vi "UHR-Fleezers Control (host) - 12.7d.vi"() -> ()   [LabVIEW 2012] (continued)
            n859 = Multiply(x="Volume (uL) P3", y=w1280) -> (x*y=w1279:dbl)
            n860 = Concatenate Strings("tvolume  " ("string"), w1287, " u" ("string"), "\r") -> (w1285:string)
            n861 = Multiply(x=w1279, y=60.0) -> (x*y=→"HP3 Flush Time (s)":dbl)
            n862 = VISA Write(VISA resource name=w1296, write buffer=w1285) -> (VISA resource name out=w1284:refnum<visa-resource-name>)  [unwired: 1 in, 2 out]
            n863 = Concatenate Strings("cvolume" ("string"), "\r") -> (w1283:string)
            n864 = VISA Write(VISA resource name=w1284, write buffer=w1283) -> (VISA resource name out=w1294:refnum<visa-resource-name>)  [unwired: 1 in, 2 out]
            n865 = Concatenate Strings("irun" ("string"), "\r") -> (w1292:string)
            n866 = VISA Write(VISA resource name=w1294, write buffer=w1292) -> ()  [unwired: 1 in, 3 out]
          }
          frame #1 {
            "Flushing P3" <- TRUE ("Flushing P3")
          }
        }
      }
      event "Flush Pump 1": Value Change {
        n867 = event-data() -> ()  [unwired: 7 out]
        n868 = flat-sequence {
          tunnel: [w1314] -> w1304
          tunnel: w1303 -> [w1307]
          tunnel: w1304 -> [_]
          frame #0 {
            # "set paramaters (rate, volume) for flush, clear volume"
            n869 = local write "Inject Pump 1"(TRUE ("Inject Pump 1")) -> ()
            n870 = Number To Decimal String(number="Flush rate (uL/m) P1") -> (decimal integer string=w1330:string)  [unwired: 1 in]
            n871 = Concatenate Strings("irate  " ("string"), w1330, " u/m" ("string"), "\r") -> (w1332:string)
            n872 = VISA Write(VISA resource name=w1307, write buffer=w1332) -> (VISA resource name out=w1328:refnum<visa-resource-name>)  [unwired: 1 in, 2 out]
            n873 = Reciprocal(x="Flush rate (uL/m) P1") -> (1/x=w1311:dbl)
            n874 = Number To Decimal String(number="Volume (uL) P1") -> (decimal integer string=w1319:string)  [unwired: 1 in]
            n875 = Multiply(x="Volume (uL) P1", y=w1311) -> (x*y=w1310:dbl)
            n876 = Concatenate Strings("tvolume  " ("string"), w1319, " u" ("string"), "\r") -> (w1317:string)
            n877 = Multiply(x=w1310, y=60.0) -> (x*y=→"HP1 Flush Time (s)":dbl)
            n878 = VISA Write(VISA resource name=w1328, write buffer=w1317) -> (VISA resource name out=w1316:refnum<visa-resource-name>)  [unwired: 1 in, 2 out]
            n879 = Concatenate Strings("cvolume" ("string"), "\r") -> (w1315:string)
            n880 = VISA Write(VISA resource name=w1316, write buffer=w1315) -> (VISA resource name out=w1326:refnum<visa-resource-name>)  [unwired: 1 in, 2 out]
            n881 = Concatenate Strings("irun" ("string"), "\r") -> (w1324:string)
            n882 = VISA Write(VISA resource name=w1326, write buffer=w1324) -> (VISA resource name out=w1314:refnum<visa-resource-name>)  [unwired: 1 in, 2 out]
          }
          frame #1 {
            "Flushing P1" <- TRUE ("Flushing P3")
          }
        }
      }
      event "Clear Volume": Value Change {
        n883 = event-data() -> ()  [unwired: 7 out]
        n884 = Concatenate Strings("cvolume" ("string"), "\r") -> (w1336:string)
        n885 = VISA Write(VISA resource name=w1335, write buffer=w1336) -> ()  [unwired: 1 in, 3 out]
      }
      event "Clear Volume P3": Value Change {
        n886 = event-data() -> ()  [unwired: 7 out]
        n887 = Concatenate Strings("cvolume" ("string"), "\r") -> (w1342:string)
        n888 = VISA Write(VISA resource name=w1341, write buffer=w1342) -> ()  [unwired: 1 in, 3 out]
        n889 = local write "Clear Volume P3"(FALSE ("Clear Volume P3")) -> ()
      }
      event "Clear Volume P1": Value Change {
        n890 = event-data() -> ()  [unwired: 7 out]
        n891 = Concatenate Strings("cvolume" ("string"), "\r") -> (w1347:string)
        n892 = local write "Clear Volume P1"(FALSE ("Clear Volume P1")) -> ()
        n893 = VISA Write(VISA resource name=w1346, write buffer=w1347) -> ()  [unwired: 1 in, 3 out]
      }
      event "Display On P3": Value Change {
        n894 = event-data() -> ()  [unwired: 7 out]
        n895 = Select(t="dim 100", s="Display On P3", f="dim 0") -> (s? t:f=w1353:string)
        n896 = Concatenate Strings(w1353, "\r") -> (w1355:string)
        n897 = VISA Write(VISA resource name=w1350, write buffer=w1355) -> ()  [unwired: 1 in, 3 out]
      }
      event "Display On P1": Value Change {
        n898 = event-data() -> ()  [unwired: 7 out]
        n899 = Select(t="dim 100", s="Display On P1", f="dim 0") -> (s? t:f=w1360:string)
        n900 = Concatenate Strings(w1360, "\r") -> (w1362:string)
        n901 = VISA Write(VISA resource name=w1357, write buffer=w1362) -> ()  [unwired: 1 in, 3 out]
      }
      event "Retract Pump 3": Value Change {
        n902 = event-data() -> ()  [unwired: 7 out]
        n903 = local write "Retract Pump 3"(FALSE ("Retract Pump 3")) -> ()
        n904 = case shown="True" "Retract Pump 3" {
          tunnel: w1364 -> [_ w1367]
          frame False {
          }
          frame True {
            n905 = Number To Decimal String(number="Retract Rate (uL/m)") -> (decimal integer string=w1385:string)  [unwired: 1 in]
            n906 = Concatenate Strings("wrate  " ("string"), w1385, " u/m" ("string"), "\r") -> (w1387:string)
            n907 = VISA Write(VISA resource name=w1367, write buffer=w1387) -> (VISA resource name out=w1378:refnum<visa-resource-name>)  [unwired: 1 in, 2 out]
            n908 = Number To Decimal String(number="Retract Vol 3 (uL)") -> (decimal integer string=w1380:string)  [unwired: 1 in]
            n909 = Concatenate Strings("tvolume  " ("string"), w1380, " u" ("string"), "\r") -> (w1377:string)
            n910 = VISA Write(VISA resource name=w1378, write buffer=w1377) -> (VISA resource name out=w1373:refnum<visa-resource-name>)  [unwired: 1 in, 2 out]
            n911 = Concatenate Strings("cvolume" ("string"), "\r") -> (w1374:string)
            n912 = VISA Write(VISA resource name=w1373, write buffer=w1374) -> (VISA resource name out=w1368:refnum<visa-resource-name>)  [unwired: 1 in, 2 out]
            n913 = Concatenate Strings("wrun" ("string"), "\r") -> (w1369:string)
            n914 = VISA Write(VISA resource name=w1368, write buffer=w1369) -> ()  [unwired: 1 in, 3 out]
          }
        }
      }
      event "Retract Pump 1": Value Change {
        n915 = event-data() -> ()  [unwired: 7 out]
        n916 = local write "Retract Pump 1"(FALSE ("Retract Pump 1")) -> ()
        n917 = case shown="True" "Retract Pump 1" {
          tunnel: w1389 -> [_ w1394]
          frame False {
          }
          frame True {
            n918 = local read "Retract Rate (uL/m)"() -> (w1392:dbl)
            n919 = Number To Decimal String(number=w1392) -> (decimal integer string=w1410:string)  [unwired: 1 in]
            n920 = Concatenate Strings("wrate  " ("string"), w1410, " u/m" ("string"), "\r") -> (w1412:string)
            n921 = VISA Write(VISA resource name=w1394, write buffer=w1412) -> (VISA resource name out=w1404:refnum<visa-resource-name>)  [unwired: 1 in, 2 out]
            n922 = Number To Decimal String(number="Retract Vol 1 (uL)") -> (decimal integer string=w1406:string)  [unwired: 1 in]
            n923 = Concatenate Strings("tvolume  " ("string"), w1406, " u" ("string"), "\r") -> (w1403:string)
            n924 = VISA Write(VISA resource name=w1404, write buffer=w1403) -> (VISA resource name out=w1400:refnum<visa-resource-name>)  [unwired: 1 in, 2 out]
            n925 = Concatenate Strings("cvolume" ("string"), "\r") -> (w1401:string)
            n926 = VISA Write(VISA resource name=w1400, write buffer=w1401) -> (VISA resource name out=w1395:refnum<visa-resource-name>)  [unwired: 1 in, 2 out]
            n927 = Concatenate Strings("wrun" ("string"), "\r") -> (w1396:string)
            n928 = VISA Write(VISA resource name=w1395, write buffer=w1396) -> ()  [unwired: 1 in, 3 out]
          }
        }
      }
      event "Flip Green Filter": Value Change {
        n929 = event-data() -> ()  [unwired: 7 out]
        n930 = Not(x="Flip Green Filter") -> (.not. x?=w1415:bool)
        n931 = local write "Flip Green Filter"(w1415) -> ()
        n932 = flat-sequence {
          tunnel: [w1424] -> w1420
          tunnel: [w1423] -> w1419
          tunnel: w1414 -> [w1422]
          tunnel: [w1427] -> w1418
          tunnel: w1420 -> [w1427]
          tunnel: [w1426] -> w1417
          tunnel: w1419 -> [w1426]
          tunnel: w1418 -> [w1431]
          tunnel: w1417 -> [w1430]
          tunnel: [w1429] -> w1421
          frame #0 {
            n933 = xnode "Read/Write Control"("FPGA VI Reference In"=w1422, "Green Filter Flipper"=TRUE) -> ("FPGA VI Reference Out"=w1424:T20, "error out"=w1423:errorcluster)  [unwired: 1 in]
          }
          frame #1 {
            n934 = Wait (ms)(milliseconds to wait=u32 100) -> ()  [unwired: 1 out]
          }
          frame #2 {
            n935 = xnode "Read/Write Control"("FPGA VI Reference In"=w1431, "error in"=w1430, "Green Filter Flipper"=FALSE) -> ("error out"=w1429:errorcluster)  [unwired: 1 out]
          }
        }
      }
      event "Pump 1 contents", "Pump 3 contents": Value Change {
        n936 = event-data() -> ()  [unwired: 7 out]
        n937 = local read "Pump 1 contents"() -> (→"Pump 1 cont disp":string)
        n938 = local read "Pump 3 contents"() -> (→"Pump 3 cont disp":string)
      }
      event "Reset Trap Pos. FB": Value Change {
        n939 = event-data() -> ()  [unwired: 7 out]
        n940 = xnode "Read/Write Control"("FPGA VI Reference In"=w1435, "Trap Pos. FB Reset"="Reset Trap Pos. FB") -> ()  [unwired: 1 in, 2 out]
      }
      event "Rem fb disp offset": Value Change {
        n941 = event-data() -> ()  [unwired: 7 out]
        n942 = local write "Rem fb disp offset"(FALSE ("Rem fb disp offset")) -> ()
        n943 = local read "Mean T1 Position (nm)"() -> (w1438:dbl)
        n944 = local read "FB Trap Pos Offset"() -> (w1439:dbl)
        n945 = Subtract(x=w1439, y=w1438) -> (x-y=w1437:dbl)
        n946 = local write "FB Trap Pos Offset"(w1437) -> ()
      }
      event "Threshold (nm)": Value Change {
        n947 = event-data() -> ()  [unwired: 7 out]
        n948 = flat-sequence {
          tunnel: [w1444] -> w1442
          tunnel: w1441 -> [w1443]
          tunnel: w1442 -> [w1455]
          frame #0 {
            n949 = xnode "Read/Write Control"("FPGA VI Reference In"=w1443) -> ("FPGA VI Reference Out"=w1447:T20, "error out"=w1446:errorcluster, "FPGA TTrig Thresh"=w1448:i64)  [unwired: 1 in]
            n950 = local read "Threshold stored (nm)"() -> (w1454:dbl)
            n951 = local read "Threshold (nm)"() -> (w1444:dbl)
            n952 = local read "AOM X Cal (nm/MHz)"() -> (w1452:dbl)
            n953 = Subtract(x=w1444, y=w1454) -> (x-y=w1453:dbl)
            n954 = Divide(x=w1453, y=w1452) -> (x/y=w1450:dbl)
            n955 = call "IR AOM freq to word.vi"("Frequency In (MHz)"=w1450) -> ("Frequency Word Out (double)"=w1451:dbl)
            n956 = To Quad Integer(1:w1451) -> (0:w1449:i64)
            n957 = Add(x=w1448, y=w1449) -> (x+y=w1445:i64)
            n958 = xnode "Read/Write Control"("FPGA VI Reference In"=w1447, "error in"=w1446, "FPGA TTrig Thresh"=w1445) -> ()  [unwired: 2 out]
          }
          frame #1 {
            "Threshold stored (nm)" <- w1455
          }
        }
      }
      event "FB Trig Integrate": Value Change {
        n959 = event-data() -> ()  [unwired: 7 out]
        n960 = local read "FB Trig Integrate"() -> (w1458:u32)
        n961 = xnode "Read/Write Control"("FPGA VI Reference In"=w1456, "FB Trig Integrate"=w1458) -> ("error out"=w1457:errorcluster)  [unwired: 1 in, 1 out]
      }
      event "11": Value Change {
        n962 = event-data() -> ()  [unwired: 7 out]
        n963 = local read "11"() -> (w1459:bool)
        n964 = case shown="True" w1459 {
          frame False {
          }
          frame True {
            n965 = local read "Messages"() -> (w1461:string)
            n966 = call "Update messages.vi"("Message to add"="You kicked it up to 11!", "Old message string"=w1461) -> ("New message string"=w1462:string)
            n967 = call <vilib>:"Beep.vi"() -> ()  [unwired: 12 in]
            n968 = local write "Messages"(w1462) -> ()
          }
        }
      }
      event "Trap Pos. FB ON": Value Change {
        n969 = event-data() -> ()  [unwired: 7 out]
        n970 = xnode "Read/Write Control"("FPGA VI Reference In"=w1463, "Force feedback"="Trap Pos. FB ON") -> ()  [unwired: 1 in, 2 out]
      }
      event "Remove Action Offset": Value Change {
        n971 = event-data() -> ()  [unwired: 7 out]
        n972 = local write "Remove Action Offset"(FALSE ("Remove Action Offset")) -> ()
        n973 = local read "Trap Pos. FB Mult Factor"() -> (w1470:i64)
        n974 = local read "Trap Pos FB Action"() -> (w1468:i64)
        n975 = local read "Trap Pos. FB Offset Factor"() -> (w1466:i64)
        n976 = Multiply(x=w1470, y=w1468) -> (x*y=w1469:i64)
        n977 = Add(x=w1469, y=w1466) -> (x+y=w1467:i64)
        n978 = local write "Trap Pos. FB Offset Factor"(w1467) -> ()
        n979 = xnode "Read/Write Control"("FPGA VI Reference In"=w1465, "Trap Pos. FB Offset Factor"=w1467) -> ()  [unwired: 1 in, 2 out]
      }
      event "Remove Unwinding Offset": Value Change {
        n980 = event-data() -> ()  [unwired: 7 out]
        n981 = local write "Remove Unwinding Offset"(FALSE ("Remove Action Offset")) -> ()
        n982 = local read "Trap Pos. FB Mult Factor"() -> (w1484:i64)
        n983 = local read "Trap Pos FB Action"() -> (w1482:i64)
        n984 = local read "Trap Pos. FB Offset Factor"() -> (w1481:i64)
        n985 = Multiply(x=w1484, y=w1482) -> (x*y=w1483:i64)
        n986 = local read "Trap Pos. FB Mult Factor"() -> (w1480:i64)
        n987 = Add(x=w1483, y=w1481) -> (x+y=w1474:i64)
        n988 = Multiply(x=32768, y="factor") -> (x*y=w1477:dbl)
        n989 = Multiply(x=w1477, y=w1480) -> (x*y=w1479:dbl)
        n990 = Subtract(x=w1474, y=w1479) -> (x-y=w1478:dbl)
        n991 = To Quad Integer(1:w1478) -> (0:w1473:i64)
        n992 = xnode "Read/Write Control"("FPGA VI Reference In"=w1472, "Trap Pos. FB Offset Factor"=w1473) -> ()  [unwired: 1 in, 2 out]
        n993 = local write "Trap Pos. FB Offset Factor"(w1473) -> ()
      }
      event "Trap Pos. FB Range", "Trap Pos. FB Gains", "Trap Pos. FB Mult Factor", "Trap Pos. FB Offset Factor", "Trap Pos FB Negate Action", "Trap Pos FB Monitor\nT1 or T2", "Differential FB?", "Negate Diff?": Value Change {
        n994 = event-data() -> ()  [unwired: 7 out]
        n995 = Unbundle By Name("Trap Pos. FB Gains") -> ("proportional gain (Kc)"=w1489:fxp<+/-,16,8>, "integral gain (Kc*Ts/Ti)"=w1488:fxp<+/-,16,8>, "derivative gain (Kc*Td/Ts)"=w1487:fxp<+/-,16,8>)
        n996 = local read "Negate Diff?"() -> (w1494:bool)
        n997 = Unbundle By Name("Trap Pos. FB Range") -> ("output high"=w1492:fxp<+/-,16,1>, "output low"=w1491:fxp<+/-,16,1>)
        n998 = xnode "Read/Write Control"("FPGA VI Reference In"=w1486, "FB2 output high"=w1492, "FB2 output low"=w1491, "P2"=w1489, "I2"=w1488, "D2"=w1487, "Trap Pos. FB Mult Factor"="Trap Pos. FB Mult Factor", "Trap Pos. FB Offset Factor"="Trap Pos. FB Offset Factor", "Trap Pos FB Negate Action"="Trap Pos FB Negate Action", "Trap Pos FB Monitor T1 or T2"="Trap Pos FB Monitor\nT1 or T2", "AI1 X Scale"="Trap Pos. AI1 X Pre-scale", "Negate Diff?"=w1494, "Diff FB Measurement?"="Differential FB?") -> ()  [unwired: 1 in, 2 out]
      }
      event "Trap Pos FB SP", "Trap Pos FB SP 2", "Use SP 2": Value Change {
        n999 = event-data() -> ()  [unwired: 7 out]
        n1000 = Select(t="Trap Pos FB SP 2", s="Use SP 2", f="Trap Pos FB SP") -> (s? t:f=w1502:fxp<+/-,16,1>)
        n1001 = xnode "Read/Write Control"("FPGA VI Reference In"=w1501, "Trap Pos. FB SP"=w1502) -> ()  [unwired: 1 in, 2 out]
      }
      event "Offset SP2 from SP1": Value Change {
        n1002 = event-data() -> ()  [unwired: 7 out]
        n1003 = local read "Trap Pos FB SP"() -> (w1508:fxp<+/-,16,1>)
        n1004 = Add(x=w1508, y="SP2 Offset") -> (x+y=w1506:fxp<+/-,16,1>)
        n1005 = property on="Trap Pos FB SP 2" class="DigNum (strict)"("Val(Sgnl)"=w1506) -> ()  [unwired: 2 in, 2 out]
        n1006 = local write "Offset SP2 from SP1"(FALSE ("Offset SP2 from SP1")) -> ()
      }
      event "Set Reading to\nSetpoint": Value Change {
        # "This is the actual PID input signal"
        n1007 = event-data() -> ()  [unwired: 7 out]
        n1008 = local write "Set Reading to\nSetpoint"(FALSE ("Set SP to Reading")) -> ()
        n1009 = xnode "Read/Write Control"("FPGA VI Reference In"=w1510) -> ("FPGA VI Reference Out"=w1513:T20, "error out"=w1512:errorcluster, "Trap Pos FB Int-Norm Signal"=w1511:fxp<+/-,16,1>)  [unwired: 1 in]
        n1010 = local read "Differential FB?"() -> (w1514:bool)
        n1011 = case shown="False" w1514 {
          tunnel: [w1519 w1526] -> w1516
          tunnel: w1511 -> [w1517 w1526]
          frame False {
            n1012 = local read "Trap Pos FB Monitor\nT1 or T2"() -> (w1522:bool)
            n1013 = local read "Trap X AI1 (DMA)"() -> (w1525:T13)
            n1014 = Unbundle By Name(w1525) -> ("Set 1"=w1524:fxp<+/-,16,1>, "Set 2"=w1523:fxp<+/-,16,1>)
            n1015 = Select(t=w1524, s=w1522, f=w1523) -> (s? t:f=w1521:fxp<+/-,16,1>)
            n1016 = Not(x="Set SP Using...") -> (.not. x?=w1518:bool)
            n1017 = Select(t=w1517, s=w1518, f=w1521) -> (s? t:f=w1519:fxp<+/-,16,1>)
          }
          frame True {
          }
        }
        n1018 = xnode "Read/Write Control"("FPGA VI Reference In"=w1513, "error in"=w1512, "Trap Pos. FB SP"=w1516) -> ()  [unwired: 2 out]
        n1019 = local write "Trap Pos FB SP"(w1516) -> ()
      }
      event "Trap Pos. FB Out Scale 2^n": Value Change {
        n1020 = event-data() -> ()  [unwired: 7 out]
        n1021 = Scale By Power Of 2(n="Trap Pos. FB Out Scale 2^n", x=ext 1.0) -> (x*2^n=w1527:ext)
        n1022 = property on="Trap Pos. FB Mult Factor" class="DigNum (strict)"("Val(Sgnl)"=w1527) -> ()  [unwired: 2 in, 2 out]
      }
      event "Trap Pos FB Int Count": Value Change {
        n1023 = event-data() -> ()  [unwired: 7 out]
        n1024 = xnode "Read/Write Control"("FPGA VI Reference In"=w1530, "Trap Pos FB Int Count"="Trap Pos FB Int Count") -> ()  [unwired: 1 in, 2 out]
      }
      event "Trap pos": Value Change {
        n1025 = event-data() -> ()  [unwired: 7 out]
        n1026 = case shown="True" "Trap pos" {
          frame False {
            n1027 = property on="Trap Delta Graph" class="WFGraph (strict)"("Visible"=TRUE) -> ()  [unwired: 2 in, 2 out]
            n1028 = property on="Saved trap pos" class="WFGraph (strict)"("Visible"=FALSE) -> ()  [unwired: 2 in, 2 out]
          }
          frame True {
            n1029 = property on="Saved trap pos" class="WFGraph (strict)"("Visible"=TRUE) -> ()  [unwired: 2 in, 2 out]
            n1030 = property on="Trap Delta Graph" class="WFGraph (strict)"("Visible"=FALSE) -> ()  [unwired: 2 in, 2 out]
          }
        }
      }
    }
    "error out 2" <- w398
    n1031 = node-c288() -> ()  [unwired: 2 out]
  }
  n1032 = timed-loop "Rough control of MCL mirror stage (debugging)" {
    tunnel: [w1539] -> w76
    timing: w22 -> [_]
    timing-out: [_] -> w21
    tunnel: w5 -> [w1537]
    stop <- w1539 stop-if-true
    n1033 = node-c288() -> ()  [unwired: 2 out]
    n1034 = case shown="2" "MCL Mode" {
      tunnel: w1537 -> [_ w1542 w1589]
      frame 0, Default {
      }
      frame 1 {
        n1035 = node-c288() -> (w1544:T23)  [unwired: 4 out]
        n1036 = timed-loop "Oscillate MCL mirror" {
          timing: w1544 -> [_]
          timing-out: [_] -> w1543
          tunnel: w1542 -> [w1545]
          i -> [w1583]
          stop <- w1546 stop-if-true
          n1037 = node-c288() -> (w1582:i64)  [unwired: 1 out]
          n1038 = Multiply(x="AO1", y=32767.0) -> (x*y=w1578:dbl)
          n1039 = Multiply(x="AO2", y=32767.0) -> (x*y=w1573:dbl)
          n1040 = Divide(x=w1578, y=10.0) -> (x/y=w1579:dbl)
          n1041 = Divide(x=w1573, y=10.0) -> (x/y=w1574:dbl)
          n1042 = To Word Integer(number=w1579) -> (16bit integer=w1571:i16)
          n1043 = To Word Integer(number=w1574) -> (16bit integer=w1570:i16)
          n1044 = Divide(x=w1582, y=i64 1000) -> (x/y=w1553:dbl)
          n1045 = Multiply(x=w1553, y=w1583) -> (x*y=w1564:dbl)
          n1046 = Multiply(x="Osc. freq. (Hz) 2", y=6.283185307179586) -> (x*y=w1565:dbl)
          n1047 = Multiply(x=w1565, y=w1564) -> (x*y=w1563:dbl)
          n1048 = Sine(x=w1563) -> (sin(x)=w1562:dbl)
          n1049 = Multiply(x=w1562, y="Osc. amp. (V)") -> (x*y=w1560:dbl)
          n1050 = Add(x=w1560, y="Osc. center (V)") -> (x+y=w1558:dbl)
          n1051 = Divide(x=w1558, y=10.0) -> (x/y=w1556:dbl)
          n1052 = Multiply(x=w1556, y=32767.0) -> (x*y=w1551:dbl)
          n1053 = Select(t=w1551, s="Scan axis", f=w1571) -> (s? t:f=w1569:dbl)
          n1054 = Select(t=w1570, s="Scan axis", f=w1551) -> (s? t:f=w1568:dbl)
          n1055 = local read "MCL Mode"() -> (w1550:u16)
          n1056 = Not Equal?(x=w1550, y=u16 1) -> (x != y?=w1547:bool)
          n1057 = local read "Stop All"() -> (w1548:bool)
          n1058 = xnode "Read/Write Control"("FPGA VI Reference In"=w1545, "AO1"=w1569, "AO2"=w1568) -> ()  [unwired: 1 in, 2 out]
          n1059 = Compound Arithmetic op=OR(w1548, w1547) -> (w1546:bool)
          n1060 = node-c288() -> ()  [unwired: 2 out]
        }
        n1061 = node-c288(w1543) -> ()  [unwired: 1 out]
      }
      frame 2 {
        n1062 = case shown="True" "Start Scan" {
          tunnel: w1589 -> [_ w1591]
          frame False {
          }
          frame True {
            n1063 = Subtract(x="End (V)", y="Begin (V)") -> (x-y=w1598:dbl)
            n1064 = Decrement(x="N Points") -> (x-1=w1597:dbl)
            n1065 = Divide(x=w1598, y=w1597) -> (x/y=w1595:dbl)
            n1066 = for {
              N: "N Points" -> [_]
              tunnel: "Begin (V)" -> [w1614]
              tunnel: [w1606] -> w1601 mode=indexing
              tunnel: w1595 -> [w1605]
              tunnel: [w1603] -> w1594 mode=indexing
              tunnel: w1591 -> [w1602]
              i -> [w1613]
              n1067 = Multiply(x=w1605, y=w1613) -> (x*y=w1612:dbl)
              n1068 = Add(x=w1614, y=w1612) -> (x+y=w1609:dbl)
              n1069 = local read "Scan axis"() -> (w1604:bool)
              n1070 = local read "AO1"() -> (w1611:dbl)
              n1071 = local read "AO2"() -> (w1610:dbl)
              n1072 = Select(t=w1609, s=w1604, f=w1611) -> (s? t:f=w1608:dbl)
              n1073 = Select(t=w1610, s=w1604, f=w1609) -> (s? t:f=w1607:dbl)
              n1074 = flat-sequence {
                tunnel: w1608 -> [w1618]
                tunnel: w1607 -> [w1617]
                tunnel: w1602 -> [w1615]
                tunnel: [w1628] -> w1606
                tunnel: [w1627] -> w1603
                frame #0 {
                  w1621 = 10.0 ("y")
                  w1616 = 32767.0 ("y")
                  n1075 = Multiply(x=w1618, y=w1616) -> (x*y=w1624:dbl)
                  n1076 = Multiply(x=w1617, y=w1616) -> (x*y=w1622:dbl)
                  n1077 = Divide(x=w1624, y=w1621) -> (x/y=w1625:dbl)
                  n1078 = Divide(x=w1622, y=w1621) -> (x/y=w1623:dbl)
                  n1079 = To Word Integer(number=w1625) -> (16bit integer=w1619:i16)
                  n1080 = To Word Integer(number=w1623) -> (16bit integer=w1620:i16)
                  n1081 = xnode "Read/Write Control"("FPGA VI Reference In"=w1615, "AO1"=w1619, "AO2"=w1620) -> ()  [unwired: 1 in, 2 out]
                }
                frame #1 {
                  n1082 = Wait (ms)(milliseconds to wait="DAQ Delay (ms)") -> ()  [unwired: 1 out]
                }
                frame #2 {
                  n1083 = local read "Slow mean"() -> (w1628:dbl)
                  n1084 = local read "Sigma"() -> (w1627:dbl)
                }
              }
            }
            n1085 = Bundle("Begin (V)"="Begin (V)", w1595, w1601) -> (→"MCL Scan":cluster{"Begin (V)":dbl, dbl, dbl[]})  [unwired: 1 out]
            n1086 = Bundle("Begin (V)"="Begin (V)", w1595, w1594) -> (→"MCL Scan 2":cluster{"Begin (V)":dbl, dbl, dbl[]})  [unwired: 1 out]
          }
        }
      }
    }
    n1087 = local read "Stop All"() -> (w1539:bool)
    n1088 = node-c288() -> ()  [unwired: 2 out]
  }
  n1089 = timed-loop "Run Scripts, including: stage motion" {
    tunnel: w59 -> [w1637]
    tunnel: w58 -> [w1638]
    tunnel: [w1638] -> w57
    tunnel: [w1637] -> w56
    timing: w54 -> [_]
    timing-out: [_] -> w53
    tunnel: w42 -> [w1636]
    tunnel: w43 -> [w1635]
    tunnel: w32 -> [w1632]
    tunnel: w31 -> [w1631]
    tunnel: w30 -> [w1633]
    tunnel: w29 -> [w1634]
    tunnel: w17 -> [w1630]
    tunnel: w5 -> [w1629]
    stop <- w1639 stop-if-true
    n1090 = node-c288() -> ()  [unwired: 1 in, 1 out]
    n1091 = event shown="[22] \"Move in a Circle\": Value Change" {
      selector: _ -> [_ _ _ _ _ _ _ _ _ _ _ _ _ _ _ _ _ _ _ _ _ _ _ _]
      dyn-events: _ -> [_ _ _ _ _ _ _ _ _ _ _ _ _ _ _ _ _ _ _ _ _ _ _ _]
      timeout: _ -> [_ _ _ _ _ _ _ _ _ _ _ _ _ _ _ _ _ _ _ _ _ _ _ _]
      tunnel: ["Set Position" "Move to Position" _ _ _ _ _ _ "Read Harvard" _ _ _ _ _ _ "Got ADig bead" "Force FB Data\nScript" _ "Got DNA bead" "Take Stepping Data" _ "Take Detection Laser\nImage" _ _] -> _
      tunnel: [_ _ _ _ _ _ _ _ _ _ _ _ _ _ _ _ _ _ _ _ _ _ _ w2453] -> w1639
      tunnel: w1637 -> [w1657 w1665 w1678 w1708 _ _ _ _ _ w1824 w1864 w1945 w1974 w2106 w2132 _ w2168 _ _ _ _ _ _ _]
      tunnel: w1638 -> [w1658 w1666 w1679 w1709 _ _ _ _ _ w1825 w1865 w1946 w1975 w2107 w2133 _ w2169 _ _ _ _ _ _ _]
      tunnel: w1636 -> [_ _ _ _ _ _ _ _ w1809 _ _ _ _ _ _ _ _ _ _ _ _ _ _ _]
      tunnel: w1635 -> [_ _ _ _ _ _ _ _ w1808 _ _ _ _ _ _ _ _ _ _ _ _ _ _ _]
      tunnel: w1634 -> [_ _ _ _ _ _ _ _ _ _ _ _ _ _ _ _ _ _ _ _ _ _ _ _]
      tunnel: w1633 -> [_ _ _ _ _ _ _ _ _ _ _ _ _ _ _ _ _ _ _ _ _ _ _ _]
      tunnel: w1632 -> [_ _ _ _ _ _ _ _ _ _ _ _ _ _ _ _ _ _ _ _ _ _ _ _]
      tunnel: w1631 -> [_ _ _ _ _ _ _ _ _ _ _ _ _ _ _ _ _ _ _ _ _ _ _ _]
      tunnel: w1630 -> [_ _ _ _ w1736 w1764 w1788 w1799 _ _ _ _ _ _ _ _ _ _ _ _ _ _ _ w2452]
      tunnel: w1629 -> [_ _ _ _ _ _ _ _ _ _ _ _ _ _ _ _ _ _ _ _ _ _ w2328 _]
      event "Set Position", "Set Position 2", "Set Position 3", "Set Position 4", "Set Position 5", "Set Position 1": Value Change {
        n1092 = event-data() -> ()  [unwired: 1 in, 5 out]
        n1093 = Build Array("Set Position 1", "Set Position 2", "Set Position 3", "Set Position 4", "Set Position 5") -> (w1656:bool[])
        n1094 = Boolean Array To Number(Boolean array=w1656) -> (number=w1655:u32)
        n1095 = Logarithm Base 2(1:w1655) -> (0:w1647:dbl)
        n1096 = call "Read Stage Position.vi"("error in"=w1657, "VISA resource name in"=w1658) -> ("Current Position"=w1662:cluster{dbl, dbl, dbl}, "error out"=w1661:errorcluster)  [unwired: 2 out]
        n1097 = Decrement(x="Position") -> (x-1=w1645:dbl)
        n1098 = Greater Or Equal?(x=w1647, y=0.0) -> (x >= y?=w1648:bool)
        n1099 = Cluster To Array(cluster=w1662) -> (array=w1659:dbl[])
        n1100 = local write "Stage Control Serial Error"(w1661) -> ()
        n1101 = Select(t=w1647, s=w1648, f=w1645) -> (s? t:f=w1644:dbl)
        n1102 = Increment(x=w1644) -> (x+1=w1643:dbl)
        n1103 = Build Array (concatenate)(w1643, w1659) -> (w1642:dbl[])
        n1104 = Replace Array Subset(array="Saved Stage Positions", new element=w1642, index (row)=w1644) -> (w1660:dbl[][])  [unwired: 1 in]
        n1105 = local write "Saved Stage Positions"(w1660) -> ()
      }
      event "Move to Position": Value Change {
        n1106 = event-data() -> ()  [unwired: 1 in, 5 out]
        n1107 = flat-sequence {
          tunnel: w1666 -> [w1670]
          tunnel: w1665 -> [w1669]
          frame #0 {
            n1108 = local read "Saved Stage Positions"() -> (w1672:dbl[][])
            n1109 = local read "Position"() -> (w1671:dbl)
            n1110 = local write "Stage Moving"(TRUE ("Stage Moving")) -> ()
            n1111 = call "move to saved stage position.vi"("error in"=w1669, "Stage VISA resource name in"=w1670, "Position"=w1671, "Saved Stage Positions"=w1672) -> ("error out"=w1668:errorcluster)  [unwired: 1 out]
            n1112 = local write "Stage Control Serial Error"(w1668) -> ()
          }
          frame #1 {
            n1113 = call <vilib>:"Beep.vi"() -> ()  [unwired: 3 in, 9 out]
            n1114 = local write "Stage Moving"(FALSE ("Stage Moving")) -> ()
          }
        }
      }
      event "Move Cap. 1 (DNA Bottom)": Value Change {
        n1115 = event-data() -> ()  [unwired: 1 in, 5 out]
        n1116 = local write "Move Cap. 1 (DNA Bottom)"(FALSE ("Move Cap. 1 (DNA Right)")) -> ()
        n1117 = flat-sequence {
          tunnel: w1678 -> [w1681]
          tunnel: w1679 -> [w1682]
          tunnel: [w1682] -> w1676
          tunnel: [w1681] -> w1675
          tunnel: w1676 -> [w1684]
          tunnel: w1675 -> [w1683]
          frame #0 {
            n1118 = property on="Sample Channel\nFlow" class="Bool (strict)"("Val(Sgnl)"="Cap 1 Samp Flow ON") -> ()  [unwired: 2 in, 2 out]
          }
          frame #1 {
            n1119 = local read "Saved Stage Positions"() -> (w1694:dbl[][])
            n1120 = local write "Stage Moving"(TRUE ("Stage Moving")) -> ()
            n1121 = Array Subset(array=w1694, index (row)=0 ("index"), length (row)=1 ("length"), index (col)=1 ("index"), length (col)=3 ("length")) -> (w1691:dbl[][])
            n1122 = Reshape Array(w1691, 3 ("dimension size")) -> (w1689:dbl[])
            n1123 = Array To Cluster(array=w1689) -> (cluster=w1688:cluster{"[0]":dbl, "[1]":dbl, "[2]":dbl})
            n1124 = call "Set Stage Position.vi"("Position"=w1688, "error in"=w1683, "VISA resource name in"=w1684) -> ("error out"=w1687:errorcluster)  [unwired: 2 out]
            n1125 = local write "Stage Control Serial Error"(w1687) -> ()
          }
          frame #2 {
            n1126 = local write "Stage Moving"(FALSE ("Stage Moving")) -> ()
            n1127 = case shown="True" "Cap 1 Flow ON" {
              frame False {
              }
              frame True {
                n1128 = property on="Inject Pump 1" class="Bool (strict)"("Val(Sgnl)"=TRUE ("Value (Signaling)")) -> ()  [unwired: 2 in, 2 out]
              }
            }
            n1129 = call <vilib>:"Beep.vi"() -> ()  [unwired: 3 in, 9 out]
          }
          frame #3 {
            n1130 = property on="Sample Channel\nFlow" class="Bool (strict)"("Val(Sgnl)"=FALSE ("Value (Signaling)")) -> ()  [unwired: 2 in, 2 out]
            n1131 = local read "Cap. 2 BD T1?\n(ADig T1, DNA T2)"() -> (w1701:bool)
            n1132 = case shown="True" w1701 {
              tunnel: "Cap 1 T ON" -> [w1703 w1704]
              frame False {
                n1133 = property on="Trap 1 (ON/OFF)" class="Bool (strict)"("Val(Sgnl)"=w1703) -> ()  [unwired: 2 in, 2 out]
              }
              frame True {
                n1134 = property on="Trap 2 (ON/OFF)" class="Bool (strict)"("Val(Sgnl)"=w1704) -> ()  [unwired: 2 in, 2 out]
              }
            }
            n1135 = property on="Got DNA bead" class="Bool"("Key Focus"=TRUE) -> ()  [unwired: 2 in, 2 out]
          }
        }
      }
      event "Move Cap. 2 (ADig Top)": Value Change {
        n1136 = event-data() -> ()  [unwired: 1 in, 5 out]
        n1137 = local write "Move Cap. 2 (ADig Top)"(FALSE ("Move Cap. 2 (ADig Left)")) -> ()
        n1138 = flat-sequence {
          tunnel: w1708 -> [w1711]
          tunnel: w1709 -> [w1712]
          tunnel: [w1712] -> w1706
          tunnel: [w1711] -> w1705
          tunnel: w1706 -> [w1715]
          tunnel: w1705 -> [w1714]
          frame #0 {
            n1139 = property on="Sample Channel\nFlow" class="Bool (strict)"("Val(Sgnl)"="Cap 2 Samp Flow ON") -> ()  [unwired: 2 in, 2 out]
          }
          frame #1 {
            w1713 = FALSE ("Value (Signaling)")
            n1140 = local read "Saved Stage Positions"() -> (w1725:dbl[][])
            n1141 = local write "Stage Moving"(TRUE ("Stage Moving")) -> ()
            n1142 = Array Subset(array=w1725, index (row)=1 ("index"), length (row)=1 ("length"), index (col)=1 ("index"), length (col)=3 ("length")) -> (w1722:dbl[][])
            n1143 = Reshape Array(w1722, 3 ("dimension size")) -> (w1720:dbl[])
            n1144 = property on="Trap 1 (ON/OFF)" class="Bool (strict)"("Val(Sgnl)"=w1713) -> ()  [unwired: 2 in, 2 out]
            n1145 = property on="Trap 1 (ON/OFF)" class="Bool (strict)"("Val(Sgnl)"=w1713) -> ()  [unwired: 2 in, 2 out]
            n1146 = Array To Cluster(array=w1720) -> (cluster=w1719:cluster{"[0]":dbl, "[1]":dbl, "[2]":dbl})
            n1147 = call "Set Stage Position.vi"("Position"=w1719, "error in"=w1714, "VISA resource name in"=w1715) -> ("error out"=w1718:errorcluster)  [unwired: 2 out]
            n1148 = local write "Stage Control Serial Error"(w1718) -> ()
          }
          frame #2 {
            n1149 = local write "Stage Moving"(FALSE ("Stage Moving")) -> ()
            n1150 = call <vilib>:"Beep.vi"() -> ()  [unwired: 3 in, 9 out]
            n1151 = case shown="True" "Cap 2 Flow ON" {
              frame False {
              }
              frame True {
                n1152 = property on="Inject Pump 3" class="Bool (strict)"("Val(Sgnl)"=TRUE ("Value (Signaling)")) -> ()  [unwired: 2 in, 2 out]
              }
            }
          }
          frame #3 {
            n1153 = property on="Sample Channel\nFlow" class="Bool (strict)"("Val(Sgnl)"=FALSE ("Value (Signaling)")) -> ()  [unwired: 2 in, 2 out]
            n1154 = case shown="False" "Cap. 2 BD T1?\n(ADig T1, DNA T2)" {
              tunnel: "Cap 2 T ON" -> [w1734 w1735]
              frame False {
                n1155 = property on="Trap 2 (ON/OFF)" class="Bool (strict)"("Val(Sgnl)"=w1734) -> ()  [unwired: 2 in, 2 out]
              }
              frame True {
                n1156 = property on="Trap 1 (ON/OFF)" class="Bool (strict)"("Val(Sgnl)"=w1735) -> ()  [unwired: 2 in, 2 out]
              }
            }
            n1157 = property on="Got ADig bead" class="Bool"("Key Focus"=TRUE) -> ()  [unwired: 2 in, 2 out]
          }
        }
      }
      event "Initialize Blue Laser": Value Change {
        n1158 = event-data() -> ()  [unwired: 1 in, 5 out]
        n1159 = flat-sequence {
          tunnel: w1736 -> [w1755]
          frame #0 {
            n1160 = Concatenate Strings("slmp ", "Blue Laser\nModulation\nPower (mW)") -> (w1754:string)
            n1161 = call "serial write macro.vi"("String"=w1754, "Delay (ms)"="Delay (ms)", "VISA resource name"=w1755) -> ("read buffer"=w1743:string, "error out"=w1744:errorcluster, "VISA resource name out"=w1751:refnum<visa-resource-name>)
            n1162 = local write "read blue buffer"(w1743) -> ()
            n1163 = local write "Blue Error Out"(w1744) -> ()
            n1164 = call "serial write macro.vi"("String"="sdmes 1", "Delay (ms)"="Delay (ms)", "VISA resource name"=w1751) -> ("read buffer"=w1741:string, "error out"=w1742:errorcluster, "VISA resource name out"=w1749:refnum<visa-resource-name>)
            n1165 = local write "Blue Error Out"(w1742) -> ()
            n1166 = local write "read blue buffer"(w1741) -> ()
            n1167 = call "serial write macro.vi"("String"="sames 1", "Delay (ms)"="Delay (ms)", "VISA resource name"=w1749) -> ("read buffer"=w1738:string, "error out"=w1740:errorcluster, "VISA resource name out"=w1746:refnum<visa-resource-name>)
            n1168 = local write "read blue buffer"(w1738) -> ()
            n1169 = local write "Blue Error Out"(w1740) -> ()
            n1170 = call "serial write macro.vi"("String"="l1", "Delay (ms)"="Delay (ms)", "VISA resource name"=w1746) -> ("read buffer"=w1737:string, "error out"=w1739:errorcluster)  [unwired: 1 out]
            n1171 = local write "read blue buffer"(w1737) -> ()
            n1172 = local write "Blue Error Out"(w1739) -> ()
          }
          frame #1 {
            n1173 = local write "Initialize Blue Laser"(FALSE ("Initialize")) -> ()
          }
        }
      }
      event "Blue Laser Modluation Mode": Value Change {
        # "Changes the type of modulation for the blue laser"
        n1174 = event-data() -> ()  [unwired: 1 in, 5 out]
        n1175 = case shown="\"Constant Power\"" "Blue Laser Modluation Mode" {
          tunnel: ["sdmes 1" w1773 "sdmes 1" "sdmes 0"] -> w1758
          tunnel: ["sames 1" "cp" "sames 0" "sames 1"] -> w1757
          frame "Digital + Analog", Default {
          }
          frame "Constant Power" {
            n1176 = local read "Blue Laser\nModulation\nPower (mW)"() -> (w1776:string)
            n1177 = Decimal String To Number(string=w1776) -> (number=w1772:i32)  [unwired: 2 in, 1 out]
            n1178 = Divide(x=w1772, y=1000) -> (x/y=w1770:dbl)
            n1179 = Number To Fractional String(number=w1770) -> (F-format string=w1771:string)  [unwired: 3 in]
            n1180 = Concatenate Strings("p ", w1771) -> (w1773:string)
          }
          frame "Digital Only" {
          }
          frame "Analog Only" {
          }
        }
        n1181 = local read "Delay (ms)"() -> (w1767:i32)
        n1182 = call "serial write macro.vi"("String"=w1758, "Delay (ms)"=w1767, "VISA resource name"=w1764) -> ("read buffer"=w1765:string, "error out"=w1766:errorcluster, "VISA resource name out"=w1759:refnum<visa-resource-name>)
        n1183 = local write "read blue buffer"(w1765) -> ()
        n1184 = local write "Blue Error Out"(w1766) -> ()
        n1185 = local read "Delay (ms)"() -> (w1762:i32)
        n1186 = call "serial write macro.vi"("String"=w1757, "Delay (ms)"=w1762, "VISA resource name"=w1759) -> ("read buffer"=w1760:string, "error out"=w1761:errorcluster)  [unwired: 1 out]
        n1187 = local write "Blue Error Out"(w1761) -> ()
        n1188 = local write "read blue buffer"(w1760) -> ()
      }
      event "Blue Laser\nModulation\nPower (mW)": Value Change {
        n1189 = event-data() -> ()  [unwired: 1 in, 5 out]
        n1190 = local read "Blue Laser\nModulation\nPower (mW)"() -> (w1783:string)
        n1191 = local read "Blue Laser Modluation Mode"() -> (w1784:string)
        n1192 = case shown="\"Constant Power\"" w1784 {
          tunnel: w1783 -> [w1790 w1797]
          tunnel: [w1789 w1796] -> w1782
          frame "Constant Power" {
            # "Different command to change constant power instead of modulation power"
            n1193 = Decimal String To Number(string=w1790) -> (offset past number=w1795:i32)  [unwired: 2 in, 1 out]
            n1194 = Divide(x=w1795, y=1000) -> (x/y=w1793:dbl)
            n1195 = Number To Fractional String(number=w1793) -> (F-format string=w1791:string)  [unwired: 3 in]
            n1196 = Concatenate Strings("p ", w1791) -> (w1789:string)
          }
          frame Default {
            n1197 = Concatenate Strings("slmp ", w1797) -> (w1796:string)
          }
        }
        n1198 = local read "Delay (ms)"() -> (w1787:i32)
        n1199 = call "serial write macro.vi"("String"=w1782, "Delay (ms)"=w1787, "VISA resource name"=w1788) -> ("read buffer"=w1786:string, "error out"=w1785:errorcluster)  [unwired: 1 out]
        n1200 = local write "Blue Error Out"(w1785) -> ()
        n1201 = local write "read blue buffer"(w1786) -> ()
      }
      event "Send string\nto Blue Laser": Value Change {
        n1202 = event-data() -> ()  [unwired: 1 in, 5 out]
        n1203 = flat-sequence {
          tunnel: w1799 -> [w1804]
          frame #0 {
            n1204 = local read "Delay (ms)"() -> (w1801:i32)
            n1205 = call "serial write macro.vi"("String"="command string", "Delay (ms)"=w1801, "VISA resource name"=w1804) -> ("read buffer"=w1802:string, "error out"=→"Blue Error Out":errorcluster)  [unwired: 1 out]
            "read blue buffer" <- w1802
            n1206 = String Length(string=w1802) -> (length=→"length":i32)
            "command string sent" <- "command string"
          }
          frame #1 {
            n1207 = local write "Send string\nto Blue Laser"(FALSE ("Send string")) -> ()
          }
        }
      }
      event "Read Harvard": Value Change {
        n1208 = event-data() -> ()  [unwired: 1 in, 5 out]
        n1209 = Concatenate Strings("write buffer", "\r") -> (w1811:string)
        n1210 = VISA Write(VISA resource name=w1809, write buffer=w1811, error in (no error)=w1808) -> (VISA resource name out=w1820:refnum<visa-resource-name>, error out=w1819:errorcluster)  [unwired: 1 out]
        n1211 = stacked-sequence {
          tunnel: [w1823] -> w1818
          tunnel: w1820 -> [w1823]
          tunnel: w1819 -> [w1822]
          tunnel: [w1822] -> w1813
          frame #0 {
            n1212 = Wait (ms)(milliseconds to wait=50) -> ()  [unwired: 1 out]
          }
        }
        n1213 = property class="Instr"(reference=w1818, error in=w1813) -> (reference out=w1817:refnum<visa-resource-name>, error out=w1815:errorcluster, "Serial Settings:Number of Bytes at Serial Port"=w1816:u32)
        "Serial Settings:Number of Bytes at Serial Port" <- w1816
        n1214 = VISA Read(VISA resource name=w1817, byte count=w1816, error in (no error)=w1815) -> (read buffer=w1814:string)  [unwired: 3 out]
        "read buffer" <- w1814
        n1215 = Fract/Exp String To Number(string=w1814) -> ()  [unwired: 5 out]
      }
      event "+z", "-z": Value Change {
        n1216 = event-data() -> ()  [unwired: 1 in, 5 out]
        n1217 = flat-sequence {
          tunnel: w1824 -> [w1846]
          tunnel: w1825 -> [w1826]
          frame #0 {
            n1218 = call "Read Stage Position.vi"("error in"=w1846, "VISA resource name in"=w1826) -> ("Current Position"=w1831:cluster{dbl, dbl, dbl}, "error out"=w1844:errorcluster, "VISA resource name out"=w1845:refnum<visa-resource-name>)  [unwired: 1 out]
            n1219 = local read "Saved Stage Positions"() -> (w1855:dbl[][])
            n1220 = Divide(x="z nudge increment (um)", y=1000.0) -> (x/y=w1843:dbl)
            n1221 = Boolean To (0,1)(Boolean="+z") -> (0, 1=w1835:i16)
            n1222 = Boolean To (0,1)(Boolean="-z") -> (0, 1=w1836:i16)
            n1223 = Array Subset(array=w1855, index (row)=1 ("index"), length (row)=1 ("length"), index (col)=1 ("index"), length (col)=3 ("length")) -> (w1852:dbl[][])
            n1224 = Multiply(x=w1835, y=w1843) -> (x*y=w1839:dbl)
            n1225 = Multiply(x=w1836, y=w1843) -> (x*y=w1837:dbl)
            n1226 = Unbundle(w1831) -> (w1829:dbl, w1828:dbl, w1832:dbl)
            n1227 = Negate(x=w1837) -> (-x=w1838:dbl)
            n1228 = Reshape Array(w1852, 3 ("dimension size")) -> (w1850:dbl[])
            n1229 = Add(x=w1839, y=w1838) -> (x+y=w1840:dbl)
            n1230 = Array To Cluster(array=w1850) -> ()  [unwired: 1 out]
            n1231 = Add(x=w1840, y=w1832) -> (x+y=w1830:dbl)
            n1232 = Bundle(cluster=w1831, w1829, w1828, w1830) -> (w1827:cluster{dbl, dbl, dbl})
            n1233 = call "Set Stage Position.vi"("Position"=w1827, "error in"=w1844, "VISA resource name in"=w1845) -> ("error out"=w1849:errorcluster)  [unwired: 2 out]
            n1234 = local write "Stage Moving"(TRUE ("Stage Moving")) -> ()
            n1235 = local write "Stage Control Serial Error"(w1849) -> ()
          }
          frame #1 {
            n1236 = local write "Stage Moving"(FALSE ("Stage Moving")) -> ()
            n1237 = call <vilib>:"Beep.vi"() -> ()  [unwired: 3 in, 9 out]
          }
        }
      }
      event "Cal/Data Acq. Spot": Value Change {
        n1238 = event-data() -> ()  [unwired: 1 in, 5 out]
        n1239 = flat-sequence {
          tunnel: w1864 -> [w1868]
          tunnel: w1865 -> [w1869]
          tunnel: [w1869] -> w1861
          tunnel: [w1868] -> w1860
          tunnel: w1861 -> [w1874]
          tunnel: w1860 -> [w1873]
          tunnel: ["Cal @ (MHz)"] -> w1858
          tunnel: [w1878] -> w1862
          tunnel: w1858 -> [w1878]
          tunnel: w1862 -> [w1887]
          tunnel: ["W/ Offset 1"] -> w1859
          tunnel: w1862 -> [w1908]
          tunnel: w1859 -> [w1906]
          frame #0 {
            n1240 = property on="Sample Channel\nFlow" class="Bool (strict)"("Val(Sgnl)"="Daq spot flow on") -> ()  [unwired: 2 in, 2 out]
            n1241 = Wait (ms)(milliseconds to wait=u32 250) -> ()  [unwired: 1 out]
          }
          frame #1 {
            n1242 = local read "Saved Stage Positions"() -> (w1871:dbl[][])
            n1243 = property on="Trap Delta (MHz)" class="DigNum (strict)"("Val(Sgnl)"="Cal @ (MHz)") -> ()  [unwired: 2 in, 2 out]
            n1244 = local write "Stage Moving"(TRUE ("Stage Moving")) -> ()
            n1245 = call "move to saved stage position.vi"("error in"=w1873, "Stage VISA resource name in"=w1874, "Position"="Cal Stage Position", "Saved Stage Positions"=w1871) -> ("error out"=w1872:errorcluster)  [unwired: 1 out]
            n1246 = local write "Stage Control Serial Error"(w1872) -> ()
          }
          frame #2 {
            n1247 = local write "Stage Moving"(FALSE ("Stage Moving")) -> ()
            n1248 = property on="Sample Channel\nFlow" class="Bool (strict)"("Val(Sgnl)"="Flow ON during cal?") -> ()  [unwired: 2 in, 2 out]
            n1249 = call <vilib>:"Beep.vi"() -> ()  [unwired: 3 in, 9 out]
          }
          frame #3 {
            n1250 = Wait (ms)(milliseconds to wait=u32 1000) -> ()  [unwired: 1 out]
          }
          frame #4 {
            n1251 = property on="Save Calibration" class="Bool (strict)"("Val(Sgnl)"=TRUE ("Value (Signaling)")) -> ()  [unwired: 2 in, 2 out]
          }
          frame #5 {
            n1252 = Wait (ms)(milliseconds to wait=u32 2000) -> ()  [unwired: 1 out]
          }
          frame #6 {
            # "Check to see if \nsaving done"
            n1253 = while {
              stop <- w1883 stop-if-true
              n1254 = local read "Saving..."() -> (w1884:bool)
              n1255 = Wait (ms)(milliseconds to wait=u32 100) -> ()  [unwired: 1 out]
              n1256 = Not(x=w1884) -> (.not. x?=w1883:bool)
            }
          }
          frame #7 {
            n1257 = case shown="True" "W/ Offset 1" {
              tunnel: w1887 -> [_ w1888]
              frame False {
              }
              frame True {
                n1258 = stacked-sequence {
                  tunnel: w1888 -> [_ _ _ _ _ _ _ w1905]
                  frame #0 {
                    n1259 = property on="Trap Delta (MHz)" class="DigNum (strict)"("Val(Sgnl)"="Offset 1 Start (MHz)") -> ()  [unwired: 2 in, 2 out]
                    n1260 = Replace Array Subset(array=u32[] [0] ("Index Values"), new element="Offset 1 Set", index=0) -> (w1889:u32[])
                    n1261 = property on="Saved AOD Raster Scan Parameter Sets" class="Arr (strict)"("Index Values"=w1889) -> ()  [unwired: 2 in, 2 out]
                  }
                  frame #1 {
                    n1262 = Wait (ms)(milliseconds to wait=u32 200) -> ()  [unwired: 1 out]
                  }
                  frame #2 {
                    n1263 = property on="Load parameters" class="Bool (strict)"("Val(Sgnl)"=TRUE ("Value (Signaling)")) -> ()  [unwired: 2 in, 2 out]
                  }
                  frame #3 {
                    n1264 = Wait (ms)(milliseconds to wait=u32 200) -> ()  [unwired: 1 out]
                  }
                  frame #4 {
                    n1265 = property on="Trap Raster Scan" class="Bool (strict)"("Val(Sgnl)"=TRUE ("Value (Signaling)")) -> ()  [unwired: 2 in, 2 out]
                  }
                  frame #5 {
                    n1266 = Wait (ms)(milliseconds to wait=u32 2000) -> ()  [unwired: 1 out]
                  }
                  frame #6 {
                    n1267 = while {
                      stop <- w1902 stop-if-true
                      n1268 = local read "Raster Scanning..."() -> (w1904:bool)
                      n1269 = local read "Saving..."() -> (w1900:bool)
                      n1270 = Wait (ms)(milliseconds to wait=u32 100) -> ()  [unwired: 1 out]
                      n1271 = Not(x=w1900) -> (.not. x?=w1899:bool)
                      n1272 = Not(x=w1904) -> (.not. x?=w1901:bool)
                      n1273 = And(x=w1901, y=w1899) -> (x .and. y?=w1902:bool)
                    }
                  }
                  frame #7 {
                    n1274 = property on="Trap Delta (MHz)" class="DigNum (strict)"("Val(Sgnl)"=w1905) -> ()  [unwired: 2 in, 2 out]
                  }
                }
              }
            }
          }
          frame #8 {
            n1275 = local read "Save ave N"() -> (w1907:dbl)
            n1276 = case shown="False" "W/ Offset 2" {
              tunnel: w1908 -> [_ w1915]
              tunnel: w1907 -> [_ w1914]
              tunnel: w1906 -> [w1910 _]
              frame False {
                n1277 = case shown="False" w1910 {
                  frame False {
                    n1278 = Multiply(x="Cal read wait (s)", y=u32 1000 ("milliseconds to wait")) -> (x*y=w1912:u32)
                    n1279 = Wait (ms)(milliseconds to wait=w1912) -> ()  [unwired: 1 out]
                  }
                  frame True {
                  }
                }
              }
              frame True {
                n1280 = stacked-sequence {
                  tunnel: w1915 -> [_ _ _ _ _ _ _ _ _ w1936 _ _]
                  tunnel: w1914 -> [_ _ _ _ _ _ _ _ _ w1934 _ _]
                  frame #0 {
                    n1281 = property on="Save ave N" class="DigNum (strict)"("Val(Sgnl)"=1.0 ("Value (Signaling)")) -> ()  [unwired: 2 in, 2 out]
                  }
                  frame #1 {
                    n1282 = Wait (ms)(milliseconds to wait=u32 500) -> ()  [unwired: 1 out]
                  }
                  frame #2 {
                    n1283 = property on="Trap Delta (MHz)" class="DigNum (strict)"("Val(Sgnl)"="Offset 2 Start (MHz)") -> ()  [unwired: 2 in, 2 out]
                    n1284 = Replace Array Subset(array=u32[] [0] ("Index Values"), new element="Offset 2 Set", index=0) -> (w1920:u32[])
                    n1285 = property on="Saved AOD Raster Scan Parameter Sets" class="Arr (strict)"("Index Values"=w1920) -> ()  [unwired: 2 in, 2 out]
                  }
                  frame #3 {
                    n1286 = Wait (ms)(milliseconds to wait=u32 500) -> ()  [unwired: 1 out]
                  }
                  frame #4 {
                    n1287 = property on="Load parameters" class="Bool (strict)"("Val(Sgnl)"=TRUE ("Value (Signaling)")) -> ()  [unwired: 2 in, 2 out]
                  }
                  frame #5 {
                    n1288 = Wait (ms)(milliseconds to wait=u32 500) -> ()  [unwired: 1 out]
                  }
                  frame #6 {
                    n1289 = property on="Trap Raster Scan" class="Bool (strict)"("Val(Sgnl)"=TRUE ("Value (Signaling)")) -> ()  [unwired: 2 in, 2 out]
                  }
                  frame #7 {
                    n1290 = Wait (ms)(milliseconds to wait=u32 2000) -> ()  [unwired: 1 out]
                  }
                  frame #8 {
                    n1291 = while {
                      stop <- w1929 stop-if-true
                      n1292 = local read "Raster Scanning..."() -> (w1932:bool)
                      n1293 = local read "Saving..."() -> (w1930:bool)
                      n1294 = Wait (ms)(milliseconds to wait=u32 100) -> ()  [unwired: 1 out]
                      n1295 = Not(x=w1930) -> (.not. x?=w1928:bool)
                      n1296 = Not(x=w1932) -> (.not. x?=w1931:bool)
                      n1297 = And(x=w1931, y=w1928) -> (x .and. y?=w1929:bool)
                    }
                  }
                  frame #9 {
                    n1298 = property on="Trap Delta (MHz)" class="DigNum (strict)"("Val(Sgnl)"=w1936) -> ()  [unwired: 2 in, 2 out]
                    n1299 = property on="Saved AOD Raster Scan Parameter Sets" class="Arr (strict)"("Index Values"=u32[] [0]) -> ()  [unwired: 2 in, 2 out]
                    n1300 = property on="Save ave N" class="DigNum (strict)"("Val(Sgnl)"=w1934) -> ()  [unwired: 2 in, 2 out]
                  }
                  frame #10 {
                    n1301 = Wait (ms)(milliseconds to wait=u32 500) -> ()  [unwired: 1 out]
                  }
                  frame #11 {
                    n1302 = property on="Load parameters" class="Bool (strict)"("Val(Sgnl)"=TRUE ("Value (Signaling)")) -> ()  [unwired: 2 in, 2 out]
                  }
                }
              }
            }
          }
          frame #9 {
            n1303 = property on="Read Cal" class="Bool (strict)"("Val(Sgnl)"=TRUE ("Value (Signaling)")) -> ()  [unwired: 2 in, 2 out]
          }
          frame #10 {
            n1304 = Wait (ms)(milliseconds to wait=u32 1000) -> ()  [unwired: 1 out]
          }
          frame #11 {